vi "IR Opo Main.vi"() -> ()   [LabVIEW 2016] (continued)
        n219 = invoke class="Acquisition" method="ToString"(reference=w523, error in=w522) -> (error out=w525:errorcluster, "ToString"=w524:string)  [unwired: 1 in, 1 out]
        n220 = property class="Bool"(reference=w509, "Disabled"=u8 0 ("Deaktiviert")) -> (reference out=w507:refnum<vi>, error out=w506:errorcluster)  [unwired: 1 in]
        n221 = call "uc480_Error_Handling.vi"("Error Code"=w521, "Error String"=w524, "Error In"=w525) -> ("Error Out"=w520:errorcluster)  [unwired: 8 in]
        n222 = Close Reference(reference=w507, error in (no error)=w506) -> ()  [unwired: 1 out]
        n223 = Close Reference(reference=w503, error in (no error)=w502) -> ()  [unwired: 1 out]
        n224 = Close Reference(reference=w505, error in (no error)=w504) -> ()  [unwired: 1 out]
        n225 = Get Date/Time In Seconds() -> (seconds since 1Jan1904=w497:timestamp)
        n226 = Format Date/Time String(time format string (%c)="%m/%d/%y - %I:%M %p  ", seconds (now)=w497) -> (date/time string=w496:string)  [unwired: 1 in]
        n227 = Concatenate Strings(w496, "Camera started", "\r") -> (w501:string)
        n228 = invoke on="Log" class="Str" method="Append String"("string"=w501) -> (error out=w494:errorcluster)  [unwired: 3 in, 3 out]
        n229 = property on="Log" class="Str"(error in=w494, "Text.Scroll Position"=u32 500000) -> ()  [unwired: 1 in, 2 out]
        n230 = case shown="False" w526 {
          tunnel: [w531 w541] -> w515
          tunnel: w520 -> [w537 w541]
          tunnel: w518 -> [w536 w540]
          tunnel: [w536 w540] -> w517
          frame False {
            w529 = 1 items=["IS_DONT_WAIT", "IS_WAIT"] ("Wait")
            n231 = property class="Camera"(reference=w536, error in=w537) -> (error out=w538:errorcluster, "Acquisition"=w539:refnum<k24>)  [unwired: 1 out]
            n232 = invoke class="Acquisition" method="Capture"(reference=w539, error in=w538, "param"=w529) -> (reference out=w532:refnum<k24>, error out=w533:errorcluster, "Capture"=w530:i32)  [unwired: 1 in, 1 out]
            n233 = invoke class="Acquisition" method="ToString"(reference=w532, error in=w533) -> (error out=w535:errorcluster, "ToString"=w534:string)  [unwired: 1 in, 1 out]
            n234 = call "uc480_Error_Handling.vi"("Error Code"=w530, "Error String"=w534, "Error In"=w535) -> ("Error Out"=w531:errorcluster)  [unwired: 8 in]
          }
          frame True {
          }
        }
      }
    }
    n235 = call "uc480_SubVI_Example_SyncEventLoop.vi"("Error In"=w55, "use sync"=w57, ".NET (Reference)"=w56) -> ("Error Out"=w53:errorcluster, "Synchronize (ms)"=w54:dbl)  [unwired: 7 in]
    "Error Out" <- w53
    n236 = Wait Until Next ms Multiple(millisecond multiple=w54) -> ()  [unwired: 1 out]
  }
  n237 = flat-sequence "Initialization sequence" {
    tunnel: [w548] -> w3
    tunnel: [w547] -> w2
    tunnel: [w546] -> w1
    tunnel: w3 -> [w695]
    tunnel: w2 -> [w694]
    tunnel: w1 -> [w693]
    tunnel: [w710] -> w20
    tunnel: w20 -> [w772]
    tunnel: [w755] -> w18
    tunnel: [w754] -> w17
    tunnel: [w753] -> w19
    tunnel: [w752] -> w16
    tunnel: [w751] -> w15
    tunnel: w19 -> [w783]
    tunnel: w18 -> [w782]
    tunnel: w17 -> [w781]
    tunnel: [w780] -> w14
    tunnel: w16 -> [w779]
    tunnel: w15 -> [w778]
    tunnel: [w775] -> w13
    tunnel: [w774] -> w9
    tunnel: w14 -> [w803]
    tunnel: [w803] -> w12
    tunnel: w13 -> [w802]
    tunnel: [w801] -> w10
    tunnel: w9 -> [w801]
    tunnel: w12 -> [w813]
    tunnel: [w813] -> w11
    tunnel: w10 -> [w812]
    tunnel: [w826] -> w8
    tunnel: w11 -> [w826]
    tunnel: w8 -> [w828]
    tunnel: [w828] -> w7
    tunnel: w7 -> [w830]
    tunnel: [w830] -> w6
    tunnel: w6 -> [w832]
    tunnel: [w832] -> w5
    tunnel: w5 -> [w834]
    tunnel: [w834] -> w4
    tunnel: w4 -> [w835]
    frame #0 {
      w549 = "standby" ("regular expression")
      w555 = "LASER" ("section")
      w564 = FALSE ("Visible")
      n238 = control-ref of="This VI"() -> (w565:refnum<vi>)
      n239 = control-ref of="This VI"() -> (w563:refnum<vi>)
      n240 = invoke class="VI" method="Default Vals.Reinit All"(reference=w565) -> ()  [unwired: 2 in, 3 out]
      n241 = property on="Axes Manual Control" class="Bool (strict)"("Visible"=w564) -> ()  [unwired: 2 in, 2 out]
      n242 = property on="Home Axes" class="Bool"("Visible"=w564) -> ()  [unwired: 2 in, 2 out]
      n243 = property class="VI"(reference=w563) -> ("Path"=w562:path)  [unwired: 1 in, 2 out]
      n244 = Strip Path(path=w562) -> (stripped path=w561:path)  [unwired: 1 out]
      n245 = Build Path(base path=w561, name or relative path="General_Configuration.ini") -> (appended path=w559:path)
      n246 = call <vilib>:"Open Config Data.vi"("create file if necessary (T)"=FALSE, "configuration file path"=w559) -> ("refnum"=w542:T5)  [unwired: 7 in, 2 out]
      n247 = call-poly <vilib>:"Read Key.vi"("section"=w555, "default value"="COM7", "key"="VISA", "refnum"=w542) -> ("error out"=w545:errorcluster, "value"=w547:string)  [unwired: 4 in, 2 out]
      "VISA Laser port" <- w547
      n248 = call-poly <vilib>:"Read Key.vi"("section"=w555, "default value"=400, "key"="Delay", "refnum"=w542) -> ("error out"=w544:errorcluster, "value"=w546:i32)  [unwired: 4 in, 2 out]
      "Laser Com Delay" <- w546
      n249 = call "CheckStatus.vi"("delay before read (ms)"=w546, "VISA resource name"=w547) -> ("read buffer"=w552:string)  [unwired: 6 in, 3 out]
      n250 = xnode "Match Regular Expression"("input string"=w552, "regular expression"=w549) -> ("whole match"=w550:string, "error out"=w548:errorcluster)  [unwired: 4 in, 3 out]
      n251 = Equal?(x=w550, y=w549) -> (x = y?=w551:bool)
      n252 = case shown="True" w551 {
        frame False {
        }
        frame True {
          n253 = Get Date/Time In Seconds() -> (seconds since 1Jan1904=w683:timestamp)
          n254 = Format Date/Time String(time format string (%c)="%m/%d/%y -%I:%M %p  ", seconds (now)=w683) -> (date/time string=w682:string)  [unwired: 1 in]
          n255 = Concatenate Strings(w682, "Initializing the ICE450 Ultra..." ("Initialiazation"), "\r") -> (w687:string)
          n256 = invoke on="Log" class="Str" method="Append String"("string"=w687) -> (error out=w680:errorcluster)  [unwired: 3 in, 3 out]
          n257 = property on="Log" class="Str"(error in=w680, "Text.Scroll Position"=u32 500000) -> ()  [unwired: 1 in, 2 out]
        }
      }
      n258 = Merge Errors(w545, w544) -> (w543:errorcluster)
      n259 = call <vilib>:"Close Config Data.vi"("error in (no error)"=w543, "refnum"=w542) -> ()  [unwired: 8 in, 2 out]
    }
    frame #1 {
      n260 = call "ICE450 Ultra Initialization.vi"("error in (no error)"=w695, "delay before read (ms)"=w693, "VISA resource name"=w694) -> ("Repetition rate"=w688:dbl, "Laser initialization status"=w692:string)  [unwired: 7 in]
      n261 = Concatenate Strings(w692, "\r") -> (w690:string)
      n262 = invoke on="Log" class="Str" method="Append String"("string"=w690) -> ()  [unwired: 3 in, 4 out]
      n263 = local write "Repetition\nRate (Hz)"(w688) -> ()
      n264 = property on="Log" class="Str"("Text.Scroll Position"=u32 500000) -> ()  [unwired: 2 in, 2 out]
    }
    frame #2 {
      w728 = "ROI Processing" ("section")
      w736 = "XPS" ("section")
      n265 = control-ref of="This VI"() -> (w750:refnum<vi>)
      n266 = property class="VI"(reference=w750) -> ("Path"=w748:path)  [unwired: 1 in, 2 out]
      n267 = Strip Path(path=w748) -> (stripped path=w747:path)  [unwired: 1 out]
      n268 = Build Path(base path=w747, name or relative path="General_Configuration.ini") -> (appended path=w738:path)
      n269 = call <vilib>:"Open Config Data.vi"("create file if necessary (T)"=FALSE, "configuration file path"=w738) -> ("error out"=w737:errorcluster, "refnum"=w709:T5)  [unwired: 7 in, 1 out]
      n270 = call-poly <vilib>:"Read Key.vi"("section"="Communication", "default value"="192.168.254.254", "key"="XPSPort", "refnum"=w709) -> ("error out"=w703:errorcluster, "value"=→"XPS_Address":string)  [unwired: 4 in, 2 out]
      n271 = call-poly <vilib>:"Read Key.vi"("section"=w736, "error in (no error)"=w737, "default value"=1.0, "key"="InitialVelocity", "refnum"=w709) -> ("error out"=w702:errorcluster, "value"=→"Velocity":dbl)  [unwired: 3 in, 2 out]
      n272 = call-poly <vilib>:"Read Key.vi"("section"=w736, "default value"=20.0, "key"="Acceleration", "refnum"=w709) -> ("error out"=w701:errorcluster, "value"=→"Acceleration":dbl)  [unwired: 4 in, 2 out]
      n273 = call-poly <vilib>:"Read Key.vi"("section"="Laser" ("key"), "default value"=0, "key"="Wavelenght", "refnum"=w709) -> ("error out"=w700:errorcluster, "value"=→"Default Wavelenght":i32)  [unwired: 4 in, 2 out]
      n274 = Merge Errors(w703, w702, w701, w700) -> (w704:errorcluster)
      n275 = call-poly <vilib>:"Read Key.vi"("section"=w728, "key"="Pixel Size", "refnum"=w709) -> ("error out"=w719:errorcluster, "value"=w708:dbl)  [unwired: 5 in, 2 out]
      n276 = call-poly <vilib>:"Read Key.vi"("section"=w728, "key"="Heigth step divider", "refnum"=w709) -> ("error out"=w718:errorcluster, "value"=w707:i32)  [unwired: 5 in, 2 out]
      n277 = call-poly <vilib>:"Read Key.vi"("section"=w728, "key"="Precision (%)", "refnum"=w709) -> ("error out"=w717:errorcluster, "value"=w705:dbl)  [unwired: 5 in, 2 out]
      n278 = call-poly <vilib>:"Read Key.vi"("section"=w728, "key"="Sampling speed", "refnum"=w709) -> ("error out"=w716:errorcluster, "value"=w706:i32)  [unwired: 5 in, 2 out]
      n279 = call-poly <vilib>:"Read Key.vi"("section"=w728, "key"="Width", "refnum"=w709) -> ("error out"=w715:errorcluster, "value"=w699:i32)  [unwired: 5 in, 2 out]
      n280 = call-poly <vilib>:"Read Key.vi"("section"=w728, "key"="Height", "refnum"=w709) -> ("error out"=w714:errorcluster, "value"=w698:i32)  [unwired: 5 in, 2 out]
      n281 = call-poly <vilib>:"Read Key.vi"("section"=w728, "key"="X offset", "refnum"=w709) -> ("error out"=w713:errorcluster, "value"=w697:i32)  [unwired: 5 in, 2 out]
      n282 = call-poly <vilib>:"Read Key.vi"("section"=w728, "key"="Y offset", "refnum"=w709) -> ("error out"=w712:errorcluster, "value"=w696:i32)  [unwired: 5 in, 2 out]
      n283 = Merge Errors(w719, w718, w717, w716, w715, w714, w713, w712, w704) -> (w711:errorcluster)
      n284 = local write "Height  step \ndivider"(w707) -> ()
      n285 = call <vilib>:"Close Config Data.vi"("error in (no error)"=w711, "refnum"=w709) -> ("error out"=w710:errorcluster)  [unwired: 8 in, 1 out]
      n286 = local write "Speed (µm/s)"(w706) -> ()
      n287 = local write "Precision (%)"(w705) -> ()
      n288 = local write "Pixel size"(w708) -> ()
      n289 = local write "Heigth (µm)"(w698) -> ()
      n290 = local write "Width (µm)"(w699) -> ()
      n291 = local write "Y offset"(w696) -> ()
      n292 = local write "X offset"(w697) -> ()
    }
    frame #3 {
      w756 = "\r"
      n293 = local read "XPS_Address"() -> (w773:string)
      n294 = call <userlib>:"Open TCP-IP.vi"("error in (no error)"=w772, "IP address"=w773) -> ("error out"=w770:errorcluster, "Connection ID"=w771:T6)  [unwired: 4 in, 4 out]
      n295 = call <userlib>:"Objects List Get.vi"("error in (no error)"=w770, "connection ID in"=w771) -> ("error out"=w751:errorcluster, "XPS error out"=w752:errorcluster, "connection ID out"=w753:T6, "Groups"=w769:string[])  [unwired: 4 in, 2 out]
      n296 = Get Date/Time In Seconds() -> (seconds since 1Jan1904=w765:timestamp)
      n297 = Format Date/Time String(time format string (%c)="%m/%d/%y -%I:%M %p  ", seconds (now)=w765) -> (date/time string=w758:string)  [unwired: 1 in]
      n298 = Index Array(array=w769) -> (element=w754:string)  [unwired: 1 in]
      "Axis 1" <- w754
      n299 = Index Array(array=w769, index=1) -> (element=w755:string)
      "Axis 2" <- w755
      n300 = Concatenate Strings(w758, "Axis 1: " ("Initialiazation"), w754, w756) -> (w767:string)
      n301 = Concatenate Strings(w758, "Axis 2: " ("Initialiazation"), w755, w756) -> (w759:string)
      n302 = invoke on="Log" class="Str" method="Append String"("string"=w767) -> (error out=w763:errorcluster)  [unwired: 3 in, 3 out]
      n303 = invoke on="Log" class="Str" method="Append String"("string"=w759) -> (error out=w760:errorcluster)  [unwired: 3 in, 3 out]
      n304 = property on="Log" class="Str"(error in=w763, "Text.Scroll Position"=u32 500000) -> ()  [unwired: 1 in, 2 out]
      n305 = property on="Log" class="Str"(error in=w760, "Text.Scroll Position"=u32 500000) -> ()  [unwired: 1 in, 2 out]
    }
    frame #4 {
      w797 = "Ready"
      n306 = call "Get Stages Status.vi"("error in (no error)"=w778, "XPS error in (no error)"=w779, "Group Name (250 c max)"=w781, "connection ID in"=w783) -> ("error out"=w788:errorcluster, "XPS error out"=w789:errorcluster, "Group Status String"=w785:string, "connection ID out"=w790:T6)  [unwired: 3 in, 1 out]
      n307 = call "Get Stages Status.vi"("error in (no error)"=w788, "XPS error in (no error)"=w789, "Group Name (250 c max)"=w782, "connection ID in"=w790) -> ("error out"=w786:errorcluster, "XPS error out"=w776:errorcluster, "Group Status String"=w784:string, "connection ID out"=w787:T6)  [unwired: 3 in, 1 out]
      n308 = String Subset(string=w785, offset (0)=0, length (rest)=5 ("length (rest)")) -> (substring=w795:string)
      n309 = Bundle(cluster="Axis Initial Parameters", "Velocity (units/seconds)"=5.0) -> (w799:T1)  [unwired: 3 in]
      n310 = call <userlib>:"Close TCP-IP.vi"("error in (no error)"=w786, "connection ID in"=w787) -> ("Error out"=w777:errorcluster)  [unwired: 9 in]
      n311 = local write "Axis Initial Parameters"(w799) -> ()
      n312 = String Subset(string=w784, offset (0)=0, length (rest)=5 ("length (rest)")) -> (substring=w796:string)
      n313 = call <vilib>:"Simple Error Handler.vi"("error in (no error)"=w777) -> ()  [unwired: 4 in, 5 out]
      n314 = call <vilib>:"Simple Error Handler.vi"("error in (no error)"=w776) -> ()  [unwired: 4 in, 5 out]
      n315 = Equal?(x=w795, y=w797) -> (x = y?=w775:bool)
      n316 = Equal?(x=w797, y=w796) -> (x = y?=w774:bool)
      n317 = And(x=w775, y=w774) -> (x .and. y?=w780:bool)
    }
    frame #5 {
      n318 = case shown="True" w802 {
        frame False {
        }
        frame True {
          n319 = Get Date/Time In Seconds() -> (seconds since 1Jan1904=w808:timestamp)
          n320 = Format Date/Time String(time format string (%c)="%m/%d/%y -%I:%M %p  ", seconds (now)=w808) -> (date/time string=w807:string)  [unwired: 1 in]
          n321 = Concatenate Strings(w807, "Axis 1 ready" ("Initialiazation"), "\r") -> (w805:string)
          n322 = invoke on="Log" class="Str" method="Append String"("string"=w805) -> (error out=w806:errorcluster)  [unwired: 3 in, 3 out]
          n323 = property on="Log" class="Str"(error in=w806, "Text.Scroll Position"=u32 500000) -> ()  [unwired: 1 in, 2 out]
        }
      }
    }
    frame #6 {
      n324 = case shown="True" w812 {
        frame False {
        }
        frame True {
          n325 = Get Date/Time In Seconds() -> (seconds since 1Jan1904=w818:timestamp)
          n326 = Format Date/Time String(time format string (%c)="%m/%d/%y -%I:%M %p  ", seconds (now)=w818) -> (date/time string=w817:string)  [unwired: 1 in]
          n327 = Concatenate Strings(w817, "Axis 2 ready" ("Initialiazation"), "\r") -> (w815:string)
          n328 = invoke on="Log" class="Str" method="Append String"("string"=w815) -> (error out=w816:errorcluster)  [unwired: 3 in, 3 out]
          n329 = property on="Log" class="Str"(error in=w816, "Text.Scroll Position"=u32 500000) -> ()  [unwired: 1 in, 2 out]
        }
      }
    }
    frame #7 {
      w822 = FALSE ("Visible")
      # "Set defaults"
      n330 = property on="LAMP" class="Bool (strict)"("BoolText.Text"="LAMP OFF" ("Boolean Text.Text")) -> ()  [unwired: 2 in, 2 out]
      n331 = property on="Laser Operation" class="Bool (strict)"("Blinking"=w822) -> ()  [unwired: 2 in, 2 out]
      n332 = property on="Capture" class="Bool"("Visible"=w822) -> ()  [unwired: 2 in, 2 out]
      n333 = property on="LASER" class="Bool (strict)"("BoolText.Text"="LASER OFF" ("Boolean Text.Text"), "Visible"=FALSE) -> ()  [unwired: 2 in, 2 out]
      n334 = property on="SINGLE SHOT" class="Bool"("Visible"=w822) -> ()  [unwired: 2 in, 2 out]
    }
    frame #8 {
      n335 = local write "Camera Status"("Init camera" ("Camera Status")) -> ()
    }
    frame #9 {
      n336 = Wait (ms)(milliseconds to wait=u32 1000) -> ()  [unwired: 1 out]
    }
    frame #10 {
      n337 = local write "Camera Status"("Start live") -> ()
    }
    frame #11 {
      n338 = Wait (ms)(milliseconds to wait=u32 1000) -> ()  [unwired: 1 out]
    }
    frame #12 {
      n339 = case shown="True" w835 {
        frame False {
          n340 = One Button Dialog(message="Axes not ready") -> ()  [unwired: 1 in, 1 out]
        }
        frame True {
          n341 = Get Date/Time In Seconds() -> (seconds since 1Jan1904=w842:timestamp)
          n342 = property on="Home Axes" class="Bool"("Visible"=TRUE) -> ()  [unwired: 2 in, 2 out]
          n343 = property on="Axes Manual Control" class="Bool (strict)"("Visible"=TRUE) -> ()  [unwired: 2 in, 2 out]
          n344 = Format Date/Time String(time format string (%c)="%m/%d/%y -%I:%M %p  ", seconds (now)=w842) -> (date/time string=w843:string)  [unwired: 1 in]
          n345 = Concatenate Strings(w843, "System ready" ("Initialiazation"), "\r") -> (w845:string)
          n346 = invoke on="Log" class="Str" method="Append String"("string"=w845) -> (error out=w844:errorcluster)  [unwired: 3 in, 3 out]
          n347 = property on="Log" class="Str"(error in=w844, "Text.Scroll Position"=u32 500000) -> ()  [unwired: 1 in, 2 out]
        }
      }
    }
  }
  n348 = while "Laser control & Stages Control" {
    stop <- w859 stop-if-true
    n349 = local read "Laser Com Delay"() -> (w847:i32)
    n350 = local read "VISA Laser port"() -> (w848:string)
    n351 = local read "XPS_Address"() -> (w851:string)
    n352 = local read "Axis 2"() -> (w849:string)
    n353 = local read "Axis 1"() -> (w850:string)
    n354 = event shown="[0] \"LAMP\": Value Change" {
      selector: _ -> [_ _ _ _ _ _ _ _ _ _ _ _ _ _ _ _]
      dyn-events: _ -> [_ _ _ _ _ _ _ _ _ _ _ _ _ _ _ _]
      timeout: _ -> [_ _ _ _ _ _ _ _ _ _ _ _ _ _ _ _]
      tunnel: [_ _ _ w1191 _ _ _ _ _ _ _ _ _ _ _ _] -> w859
      tunnel: [w866 w1022 w1185 _ _ _ w1246 _ w1274 w1301 _ w1376 "" ("StringOut") w1570 _ w1694] -> w852
      tunnel: w851 -> [_ _ _ _ _ _ _ _ _ w1304 _ _ w1489 w1569 _ w1681]
      tunnel: w850 -> [_ _ _ _ _ _ _ _ _ w1303 _ _ w1488 w1568 _ w1680]
      tunnel: w849 -> [_ _ _ _ _ _ _ _ _ w1302 _ _ w1487 w1567 _ w1679]
      tunnel: w848 -> [w864 w1020 w1182 w1190 _ _ w1249 w1269 _ _ _ _ _ _ _ _]
      tunnel: w847 -> [w863 w1019 w1181 w1189 _ _ w1248 w1268 _ _ _ _ _ _ _ _]
      event "LAMP": Value Change {
        n355 = event-data() -> ()  [unwired: 1 in, 6 out]
        n356 = case shown="True" "LAMP" {
          tunnel: [w867 w995] -> w866
          tunnel: w864 -> [w873 w994]
          tunnel: w863 -> [w872 w993]
          frame False {
            w868 = "standby" ("regular expression")
            n357 = call "FLStop.vi"("delay before read (ms)"=w872, "VISA resource name"=w873) -> ("read buffer"=w871:string)  [unwired: 6 in, 3 out]
            n358 = xnode "Match Regular Expression"("input string"=w871, "regular expression"=w868) -> ("whole match"=w869:string)  [unwired: 4 in, 4 out]
            n359 = Equal?(x=w869, y=w868) -> (x = y?=w870:bool)
            n360 = case shown="True" w870 {
              tunnel: ["" "Flashlamp deactivated"] -> w867
              frame False {
              }
              frame True {
                w875 = FALSE ("Visible")
                n361 = property on="LASER" class="Bool (strict)"("Visible"=w875) -> ()  [unwired: 2 in, 2 out]
                n362 = property on="Capture" class="Bool"("Visible"=w875) -> ()  [unwired: 2 in, 2 out]
                n363 = property on="SINGLE SHOT" class="Bool"("Visible"=w875) -> ()  [unwired: 2 in, 2 out]
                n364 = property on="Laser Operation" class="Bool (strict)"("Blinking"=w875) -> ()  [unwired: 2 in, 2 out]
                n365 = property on="LAMP" class="Bool (strict)"("BoolText.Text"="LAMP OFF" ("Boolean Text.Text")) -> ()  [unwired: 2 in, 2 out]
              }
            }
          }
          frame True {
            n366 = flat-sequence {
              tunnel: w994 -> [w1003]
              tunnel: w993 -> [w1002]
              tunnel: [w999] -> w992
              tunnel: [w1013] -> w995
              tunnel: w992 -> [w1012]
              frame #0 {
                w1000 = "fire" ("regular expression")
                n367 = while {
                  i -> [w1007]
                  stop <- w1010 stop-if-true
                  n368 = Wait Until Next ms Multiple(millisecond multiple=u32 1000) -> ()  [unwired: 1 out]
                  n369 = Equal?(x=5, y=w1007) -> (x = y?=w1010:bool)
                  n370 = Subtract(x=5, y=w1007) -> (x-y=w1005:i32)
                  n371 = Number To Decimal String(number=w1005) -> (decimal integer string=w1006:string)  [unwired: 1 in]
                  n372 = property on="LAMP" class="Bool (strict)"("BoolText.Text"=w1006) -> ()  [unwired: 2 in, 2 out]
                }
                n373 = Wait (ms)(milliseconds to wait=u32 5000) -> ()  [unwired: 1 out]
                n374 = call "FLStart.vi"("delay before read (ms)"=w1002, "VISA resource name"=w1003) -> ("Error Out"=w997:errorcluster, "read buffer"=w998:string)  [unwired: 6 in, 2 out]
                n375 = Match Pattern(string=w998, regular expression=w1000) -> (match substring=w1001:string)  [unwired: 1 in, 3 out]
                n376 = call <vilib>:"Simple Error Handler.vi"("error source (\" \")"="Lamp" ("error source (\" \")"), "error in (no error)"=w997) -> ()  [unwired: 3 in, 5 out]
                n377 = Equal?(x=w1001, y=w1000) -> (x = y?=w999:bool)
              }
              frame #1 {
                n378 = case shown="True" w1012 {
                  tunnel: ["Flashlamp NOT firing" "Flashlamp activated"] -> w1013
                  frame False {
                    n379 = property on="LAMP" class="Bool (strict)"("Value"=FALSE ("LAMP")) -> ()  [unwired: 2 in, 2 out]
                  }
                  frame True {
                    w1016 = TRUE ("Visible")
                    n380 = property on="LASER" class="Bool (strict)"("Visible"=w1016) -> ()  [unwired: 2 in, 2 out]
                    n381 = property on="Capture" class="Bool"("Visible"=w1016) -> ()  [unwired: 2 in, 2 out]
                    n382 = property on="LAMP" class="Bool (strict)"("BoolText.Text"="LAMP ON" ("Boolean Text.Text")) -> ()  [unwired: 2 in, 2 out]
                    n383 = property on="SINGLE SHOT" class="Bool"("Visible"=w1016) -> ()  [unwired: 2 in, 2 out]
                  }
                }
              }
            }
          }
        }
      }
      event "LASER": Value Change {
        n384 = event-data() -> ()  [unwired: 1 in, 6 out]
        n385 = case shown="False" "LASER" {
          tunnel: [w1033 w1162] -> w1023
          tunnel: [w1032 w1161] -> w1022
          tunnel: w1020 -> [w1030 w1156]
          tunnel: w1019 -> [w1029 w1155]
          frame False {
            w1027 = "fire" ("regular expression")
            n386 = local read "LAMP"() -> (w1031:bool)
            n387 = case shown="True" w1031 {
              tunnel: [FALSE ("Visible") TRUE ("Visible")] -> w1024
              frame False {
              }
              frame True {
              }
            }
            n388 = property on="Capture" class="Bool"("Visible"=w1024) -> ()  [unwired: 2 in, 2 out]
            n389 = property on="SINGLE SHOT" class="Bool"("Visible"=w1024) -> ()  [unwired: 2 in, 2 out]
            n390 = call "QSStop.vi"("delay before read (ms)"=w1029, "VISA resource name"=w1030) -> ("read buffer"=w1026:string)  [unwired: 6 in, 3 out]
            n391 = xnode "Match Regular Expression"("input string"=w1026, "regular expression"=w1027) -> ("whole match"=w1028:string)  [unwired: 4 in, 4 out]
            n392 = Equal?(x=w1028, y=w1027) -> (x = y?=w1025:bool)
            n393 = case shown="False" w1025 {
              tunnel: [FALSE w1037] -> w1033
              tunnel: ["" "Q-Switch deactivated"] -> w1032
              frame False {
              }
              frame True {
                w1037 = FALSE ("Boolean")
                n394 = property on="LASER" class="Bool (strict)"("BoolText.Text"="LASER OFF" ("Boolean Text.Text"), "Value"=w1037) -> ()  [unwired: 2 in, 2 out]
                n395 = property on="Laser Operation" class="Bool (strict)"("Blinking"=w1037) -> ()  [unwired: 2 in, 2 out]
              }
            }
          }
          frame True {
            w1158 = "fire" ("regular expression")
            n396 = call "CheckStatus.vi"("delay before read (ms)"=w1155, "VISA resource name"=w1156) -> ("read buffer"=w1160:string)  [unwired: 6 in, 3 out]
            n397 = Match Pattern(string=w1160, regular expression=w1158) -> (match substring=w1159:string)  [unwired: 1 in, 3 out]
            n398 = Equal?(x=w1159, y=w1158) -> (x = y?=w1157:bool)
            n399 = case shown="True" w1157 {
              tunnel: [FALSE ("Boolean") w1173] -> w1162
              tunnel: ["The flashlamp is not firing" w1172] -> w1161
              tunnel: w1156 -> [_ w1171]
              tunnel: w1155 -> [_ w1170]
              frame False {
                n400 = property on="LASER" class="Bool (strict)"("Value"=FALSE ("LASER")) -> ()  [unwired: 2 in, 2 out]
              }
              frame True {
                w1168 = "qs" ("regular expression")
                n401 = call "QSStart.vi"("delay before read (ms)"=w1170, "VISA resource name"=w1171) -> ("read buffer"=w1167:string)  [unwired: 6 in, 3 out]
                n402 = Match Pattern(string=w1167, regular expression=w1168) -> (match substring=w1169:string)  [unwired: 1 in, 3 out]
                n403 = Equal?(x=w1169, y=w1168) -> (x = y?=w1166:bool)
                n404 = case shown="True" w1166 {
                  tunnel: [FALSE ("Boolean") w1179] -> w1173
                  tunnel: ["Q-Switch is NOT firing" "Q-Switch activated"] -> w1172
                  frame False {
                    n405 = property on="LASER" class="Bool (strict)"("Value"=FALSE ("LASER")) -> ()  [unwired: 2 in, 2 out]
                  }
                  frame True {
                    w1177 = FALSE ("Visible")
                    w1179 = TRUE ("Boolean")
                    n406 = property on="Capture" class="Bool"("Visible"=w1177) -> ()  [unwired: 2 in, 2 out]
                    n407 = property on="Laser Operation" class="Bool (strict)"("Blinking"=w1179) -> ()  [unwired: 2 in, 2 out]
                    n408 = property on="LASER" class="Bool (strict)"("BoolText.Text"="LASER ON" ("Boolean Text.Text")) -> ()  [unwired: 2 in, 2 out]
                    n409 = property on="SINGLE SHOT" class="Bool"("Visible"=w1177) -> ()  [unwired: 2 in, 2 out]
                  }
                }
              }
            }
          }
        }
        "Laser Operation" <- w1023
      }
      event "Repetition\nRate (Hz)": Value Change {
        n410 = event-data() -> ()  [unwired: 1 in, 6 out]
        n411 = call "FLFrequencySet.vi"("Frequency (Hz)"="Repetition\nRate (Hz)", "delay before read (ms)"=w1181, "VISA resource name"=w1182) -> ()  [unwired: 5 in, 4 out]
        n412 = Number To Fractional String(number="Repetition\nRate (Hz)", precision (6)=i16 2 ("width (-)")) -> (F-format string=w1187:string)  [unwired: 2 in]
        n413 = Concatenate Strings("Repetition rate set to: " ("string"), w1187, " Hz" ("string")) -> (w1185:string)
      }
      event "EXIT": Value Change {
        n414 = event-data() -> ()  [unwired: 1 in, 6 out]
        n415 = flat-sequence {
          tunnel: w1190 -> [w1193]
          tunnel: w1189 -> [w1192]
          tunnel: ["EXIT"] -> w1191
          frame #0 {
            n416 = call "QSStop.vi"("delay before read (ms)"=w1192, "VISA resource name"=w1193) -> ("Error Out"=w1194:errorcluster)  [unwired: 6 in, 3 out]
            n417 = call "FLStop.vi"("Error In"=w1194, "delay before read (ms)"=w1192, "VISA resource name"=w1193) -> ()  [unwired: 5 in, 4 out]
          }
          frame #1 {
            n418 = Wait (ms)(milliseconds to wait=u32 1000) -> ()  [unwired: 1 out]
          }
          frame #2 {
            n419 = local write "Camera Status"("Exit camera") -> ()
          }
          frame #3 {
            n420 = Wait (ms)(milliseconds to wait=u32 1000) -> ()  [unwired: 1 out]
          }
          frame #4 {
            n421 = control-ref of="This VI"() -> (w1201:refnum<vi>)
            n422 = property class="VI"(reference=w1201) -> ("Path"=w1202:path)  [unwired: 1 in, 2 out]
            n423 = control-ref of="This Application"() -> (w1217:refnum<vi>)
            n424 = Strip Path(path=w1202) -> (stripped path=w1211:path)  [unwired: 1 out]
            n425 = property class="App"(reference=w1217) -> ("App.Kind"=w1216:T9)  [unwired: 1 in, 2 out]
            n426 = Build Path(base path=w1211, name or relative path="Logs") -> (appended path=w1209:path)
            n427 = case shown="\"Run Time System\"" w1216 {
              frame "Development System", Default {
              }
              frame "Run Time System" {
                n428 = control-ref of="This VI"() -> (w1226:refnum<vi>)
                n429 = invoke class="VI" method="FP.Close"(reference=w1226) -> ()  [unwired: 2 in, 3 out]
                n430 = Quit LabVIEW() -> ()  [unwired: 1 in]
              }
            }
            n431 = call <vilib>:"Check if File or Folder Exists.vi"("path"=w1209) -> ("file or folder exists?"=w1210:bool, "dup path"=w1212:path)  [unwired: 8 in, 1 out]
            n432 = case shown="True" w1210 {
              tunnel: w1212 -> [w1219 w1220]
              tunnel: [w1218 w1220] -> w1215
              frame False {
                n433 = Create Folder(path (use dialog)=w1219) -> (created path=w1218:path)  [unwired: 2 in, 2 out]
              }
              frame True {
              }
            }
            n434 = Get Date/Time In Seconds() -> (seconds since 1Jan1904=w1206:timestamp)
            n435 = Format Date/Time String(time format string (%c)="%d%m%y %I-%M %p ", seconds (now)=w1206) -> (date/time string=w1204:string)  [unwired: 1 in]
            n436 = Concatenate Strings(w1204, "Log File.txt") -> (w1214:string)
            n437 = Build Path(base path=w1215, name or relative path=w1214) -> (appended path=w1213:path)
            n438 = Open/Create/Replace File(file path (use dialog)=w1213, operation (0:open)=T7."replace or create") -> (refnum out=w1200:refnum<file>, cancelled=w1198:bool, error out=w1199:errorcluster)  [unwired: 4 in]
            n439 = case shown="False" w1198 {
              tunnel: w1200 -> [w1225 _]
              tunnel: w1199 -> [w1223 _]
              frame False {
                n440 = local read "Log"() -> (w1224:string)
                n441 = Write to Text File(file (use dialog)=w1225, text=w1224, error in=w1223) -> (refnum out=w1222:refnum<file>, error out=w1221:errorcluster)  [unwired: 2 out]
                n442 = Close File(refnum=w1222, error in=w1221) -> ()  [unwired: 2 out]
              }
              frame True {
              }
            }
          }
          frame #5 {
          }
        }
      }
      event "Processing time unit", "Processi time (sec)": Value Change {
        n443 = event-data() -> ()  [unwired: 1 in, 6 out]
        n444 = local read "Processing time unit"() -> (w1230:string)
        n445 = Equal?(x=w1230, y="min") -> (x = y?=w1228:bool)
        n446 = case shown="False" w1228 {
          frame False {
            n447 = local read "Processi time (sec)"() -> (w1231:i32)
            n448 = local write "Process time"(w1231) -> ()
          }
          frame True {
            n449 = local read "Processi time (sec)"() -> (w1233:i32)
            n450 = Quotient & Remainder(x=w1233, y=60) -> (floor(x/y)=w1232:i32)  [unwired: 1 out]
            n451 = local write "Process time"(w1232) -> ()
          }
        }
      }
      event "Overlay MSI Image": Value Change {
        n452 = event-data() -> ()  [unwired: 1 in, 6 out]
        n453 = vi-ref "MSI_Image_overlap.vi"() -> (w1235:refnum<vi>)
        n454 = case shown="True" "Overlay MSI Image" {
          tunnel: w1235 -> [_ w1240]
          frame False {
          }
          frame True {
            n455 = invoke class="VI" method="FP.Open"(reference=w1240, "Activate"=TRUE ("Activate?"), "State"=T8."Standard") -> (reference out=w1243:refnum<vi>, error out=w1238:errorcluster)  [unwired: 2 in, 3 out]
            n456 = invoke class="VI" method="Run VI"(reference=w1243, error in=w1238, "Wait until done"=FALSE ("Wait Until Done"), "Auto Dispose Ref"=TRUE ("Auto Dispose Reference")) -> (reference out=w1239:refnum<vi>, error out=w1237:errorcluster)  [unwired: 1 in, 3 out]
            n457 = Close Reference(reference=w1239, error in (no error)=w1237) -> ()  [unwired: 1 out]
          }
        }
      }
      event "SINGLE SHOT": Value Change {
        n458 = event-data() -> ()  [unwired: 1 in, 6 out]
        n459 = case shown="False" "SINGLE SHOT" {
          tunnel: w1249 -> [_ w1253]
          tunnel: w1248 -> [_ w1252]
          tunnel: ["" w1251] -> w1246
          frame False {
          }
          frame True {
            w1257 = "fire" ("regular expression")
            n460 = call "CheckStatus.vi"("delay before read (ms)"=w1252, "VISA resource name"=w1253) -> ("read buffer"=w1255:string)  [unwired: 6 in, 3 out]
            n461 = Match Pattern(string=w1255, regular expression=w1257) -> (match substring=w1256:string)  [unwired: 1 in, 3 out]
            n462 = Equal?(x=w1256, y=w1257) -> (x = y?=w1254:bool)
            n463 = case shown="True" w1254 {
              tunnel: ["The flashlamp is not firing" w1265] -> w1251
              tunnel: w1253 -> [_ w1264]
              tunnel: w1252 -> [_ w1263]
              frame False {
              }
              frame True {
                w1261 = "qs" ("regular expression")
                n464 = call "QSSingleShot.vi"("delay before read (ms)"=w1263, "VISA resource name"=w1264) -> ("read buffer"=w1260:string)  [unwired: 6 in, 3 out]
                n465 = Match Pattern(string=w1260, regular expression=w1261) -> (match substring=w1262:string)  [unwired: 1 in, 3 out]
                n466 = Equal?(x=w1262, y=w1261) -> (x = y?=w1259:bool)
                n467 = case shown="False" w1259 {
                  tunnel: ["Q-Switch is NOT firing" "Q-Switch activated"] -> w1265
                  frame False {
                  }
                  frame True {
                  }
                }
              }
            }
          }
        }
      }
      event "Laser Status": Value Change {
        n468 = event-data() -> ()  [unwired: 1 in, 6 out]
        n469 = case shown="True" "Laser Status" {
          tunnel: w1269 -> [_ w1272]
          tunnel: w1268 -> [_ w1271]
          frame False {
          }
          frame True {
            n470 = call "ICE450UltraMonitor.vi"("delay before read (ms)"=w1271, "VISA resource name"=w1272) -> ()  [unwired: 10 in]
          }
        }
      }
      event "Open \nManual": Value Change {
        n471 = event-data() -> ()  [unwired: 1 in, 6 out]
        n472 = case shown="True" "Open \nManual" {
          tunnel: [_ "Opening Manual" ("StringOut")] -> w1274
          frame False {
          }
          frame True {
            w1283 = FALSE  # wait until completion? (T)
            n473 = control-ref of="This VI"() -> (w1287:refnum<vi>)
            n474 = property class="VI"(reference=w1287) -> ("Path"=w1286:path)  [unwired: 1 in, 2 out]
            n475 = Strip Path(path=w1286) -> (stripped path=w1285:path)  [unwired: 1 out]
            n476 = Build Path(base path=w1285, name or relative path="LAST_Software_Manual.PDF") -> (appended path=w1277:path)
            n477 = Path To String(path=w1277) -> (string=w1280:string)
            n478 = Concatenate Strings("cmd  /c \"", w1280, "\"" ("string")) -> (w1275:string)
            n479 = call <vilib>:"System Exec.vi"("run minimized? (F)"=TRUE, "wait until completion? (T)"=w1283, "error in (no error)"="error in (no error)", "command line"=w1275) -> ("error out"=→"error out":errorcluster)  [unwired: 4 in, 3 out]
          }
        }
      }
      event "Stages status": Value Change {
        w1295 = "Ready"
        n480 = event-data() -> ()  [unwired: 1 in, 6 out]
        n481 = case shown="True" "Stages status" {
          tunnel: w1304 -> [_ w1317]
          tunnel: w1303 -> [_ w1316]
          tunnel: w1302 -> [_ w1315]
          tunnel: [w1308 w1314] -> w1301
          tunnel: [w1308 w1312] -> w1291
          tunnel: [w1308 w1313] -> w1290
          frame False {
            w1308 = ""
          }
          frame True {
            n482 = call <userlib>:"Open TCP-IP.vi"("IP address"=w1317) -> ("error out"=w1311:errorcluster, "Connection ID"=w1318:T6)  [unwired: 8 in, 1 out]
            n483 = call <vilib>:"Simple Error Handler.vi"("error in (no error)"=w1311) -> ("error?"=w1309:bool, "error out"=w1310:errorcluster)  [unwired: 4 in, 3 out]
            n484 = case shown="True" w1309 {
              tunnel: w1318 -> [w1339 _]
              tunnel: w1310 -> [w1338 _]
              tunnel: w1316 -> [w1331 _]
              tunnel: w1315 -> [w1330 _]
              tunnel: [w1329 w1340] -> w1314
              tunnel: [w1326 w1340] -> w1313
              tunnel: [w1322 w1340] -> w1312
              frame False {
                n485 = call "Get Stages Status.vi"("error in (no error)"=w1338, "Group Name (250 c max)"=w1331, "connection ID in"=w1339) -> ("error out"=w1335:errorcluster, "XPS error out"=w1334:errorcluster, "Group Status String"=w1326:string, "connection ID out"=w1337:T6)  [unwired: 4 in, 1 out]
                n486 = call "Get Stages Status.vi"("error in (no error)"=w1335, "XPS error in (no error)"=w1334, "Group Name (250 c max)"=w1330, "connection ID in"=w1337) -> ("error out"=w1332:errorcluster, "XPS error out"=w1328:errorcluster, "Group Status String"=w1322:string, "connection ID out"=w1333:T6)  [unwired: 3 in, 1 out]
                n487 = call <vilib>:"Simple Error Handler.vi"("error source (\" \")"="Stage status" ("error source (\" \")"), "error in (no error)"=w1328) -> ()  [unwired: 3 in, 5 out]
                n488 = Concatenate Strings("Axis 1 " ("string"), w1326) -> (w1325:string)
                n489 = call <userlib>:"Close TCP-IP.vi"("error in (no error)"=w1332, "connection ID in"=w1333) -> ("Error out"=w1327:errorcluster)  [unwired: 9 in]
                n490 = call <vilib>:"Simple Error Handler.vi"("error source (\" \")"="TCP close Stage status" ("error source (\" \")"), "error in (no error)"=w1327) -> ()  [unwired: 3 in, 5 out]
                n491 = Concatenate Strings("Axis 2 " ("string"), w1322) -> (w1323:string)
                n492 = Concatenate Strings(w1325, " - " ("string"), w1323) -> (w1329:string)
              }
              frame True {
                w1340 = ""
              }
            }
          }
        }
        n493 = String Subset(string=w1290, offset (0)=0, length (rest)=5 ("length (rest)")) -> (substring=w1294:string)
        n494 = String Subset(string=w1291, offset (0)=0, length (rest)=5 ("length (rest)")) -> (substring=w1296:string)
        n495 = Equal?(x=w1295, y=w1294) -> (x = y?=w1292:bool)
        n496 = Equal?(x=w1296, y=w1295) -> (x = y?=w1293:bool)
        n497 = And(x=w1293, y=w1292) -> (x .and. y?=w1289:bool)
        n498 = case shown="True" w1289 {
          frame False {
          }
          frame True {
            n499 = property on="Axes Manual Control" class="Bool (strict)"("Visible"=TRUE) -> ()  [unwired: 2 in, 2 out]
            n500 = property on="Home Axes" class="Bool"("Visible"=TRUE) -> ()  [unwired: 2 in, 2 out]
          }
        }
      }
      event "Save configuration": Value Change {
        n501 = event-data() -> ()  [unwired: 1 in, 6 out]
        n502 = case shown="True" "Save configuration" {
          frame False {
          }
          frame True {
            w1368 = "ROI Processing" ("section")
            n503 = control-ref of="This VI"() -> (w1374:refnum<vi>)
            n504 = property class="VI"(reference=w1374) -> ("Path"=w1373:path)  [unwired: 1 in, 2 out]
            n505 = Strip Path(path=w1373) -> (stripped path=w1372:path)  [unwired: 1 out]
            n506 = Build Path(base path=w1372, name or relative path="General_Configuration.ini") -> (appended path=w1370:path)
            n507 = local read "Heigth (µm)"() -> (w1354:i32)
            n508 = local read "Width (µm)"() -> (w1355:i32)
            n509 = local read "Pixel size"() -> (w1366:dbl)
            n510 = local read "X offset"() -> (w1353:i32)
            n511 = local read "Y offset"() -> (w1352:i32)
            n512 = local read "Height  step \ndivider"() -> (w1365:i32)
            n513 = call <vilib>:"Open Config Data.vi"("create file if necessary (T)"=FALSE, "configuration file path"=w1370) -> ("refnum"=w1342:T5)  [unwired: 7 in, 2 out]
            n514 = local read "Speed (µm/s)"() -> (w1356:i32)
            n515 = local read "Precision (%)"() -> (w1357:dbl)
            n516 = call-poly <vilib>:"Write Key.vi"("section"=w1368, "value"=w1366, "key"="Pixel Size", "refnum"=w1342) -> ("error out"=w1351:errorcluster)  [unwired: 5 in, 2 out]
            n517 = call-poly <vilib>:"Write Key.vi"("section"=w1368, "value"=w1365, "key"="Heigth step divider", "refnum"=w1342) -> ("error out"=w1350:errorcluster)  [unwired: 5 in, 2 out]
            n518 = call-poly <vilib>:"Write Key.vi"("section"=w1368, "value"=w1357, "key"="Precision (%)", "refnum"=w1342) -> ("error out"=w1349:errorcluster)  [unwired: 5 in, 2 out]
            n519 = call-poly <vilib>:"Write Key.vi"("section"=w1368, "value"=w1356, "key"="Sampling speed", "refnum"=w1342) -> ("error out"=w1348:errorcluster)  [unwired: 5 in, 2 out]
            n520 = call-poly <vilib>:"Write Key.vi"("section"=w1368, "value"=w1355, "key"="Width", "refnum"=w1342) -> ("error out"=w1347:errorcluster)  [unwired: 5 in, 2 out]
            n521 = call-poly <vilib>:"Write Key.vi"("section"=w1368, "value"=w1354, "key"="Height", "refnum"=w1342) -> ("error out"=w1346:errorcluster)  [unwired: 5 in, 2 out]
            n522 = call-poly <vilib>:"Write Key.vi"("section"=w1368, "value"=w1353, "key"="X offset", "refnum"=w1342) -> ("error out"=w1345:errorcluster)  [unwired: 5 in, 2 out]
            n523 = call-poly <vilib>:"Write Key.vi"("section"=w1368, "value"=w1352, "key"="Y offset", "refnum"=w1342) -> ("error out"=w1344:errorcluster)  [unwired: 5 in, 2 out]
            n524 = Merge Errors(w1351, w1350, w1349, w1348, w1347, w1346, w1345, w1344) -> (w1343:errorcluster)
            n525 = call <vilib>:"Close Config Data.vi"("error in (no error)"=w1343, "refnum"=w1342) -> ()  [unwired: 8 in, 2 out]
          }
        }
      }
      event "Process Image": Value Change {
        n526 = event-data() -> ()  [unwired: 1 in, 6 out]
        n527 = case shown="True" "Process Image" {
          tunnel: ["" "Processing done"] -> w1376
          frame False {
          }
          frame True {
            w1403 = 0.5  # Delay after laser on/off
            w1415 = 2.0 ("y")
            w1452 = T10 0 items=["Grayscale (U8)", "Grayscale (I16)", "Grayscale (SGL)", "Complex (CSG)", "RGB (U32)", "HSL (U32)", "RGB (U64)", "Grayscale (U16)"] ("Image Type")
            w1455 = i16 4 ("precision (6)")
            w1447 = 1000 ("y")
            n528 = local read "Source"() -> (w1454:T2)
            n529 = property on="Source" class="ImageControl"() -> ("ROI"=w1458:T11)  [unwired: 2 in, 2 out]
            n530 = call "IMAQ Cast Image"("Image Type"=w1452, "Image Src"=w1454) -> ("error out"=w1383:errorcluster, "Image Dst Out"=w1453:T2)  [unwired: 8 in]
            n531 = Unbundle By Name(w1458) -> ("Global Rectangle"=w1388:i32[])
            n532 = call "IMAQ ROIToMask 2"("error in (no error)"=w1383, "ROI Descriptor"=w1458, "Image"=w1453) -> ("error out"=w1384:errorcluster, "Image Out"=w1460:T2)  [unwired: 6 in, 1 out]
            n533 = call "IMAQ ImageToArray"("error in (no error)"=w1384, "Image"=w1460) -> ("error out"=w1382:errorcluster, "Image Pixels (U8)"=w1437:u8[][])  [unwired: 2 in, 3 out]
            n534 = Array To Cluster(array=w1388) -> (cluster=w1387:T12)
            n535 = local read "X offset"() -> (w1450:i32)